vi "View_series_FITS.vi"() -> ()   [LabVIEW 2017] (continued)
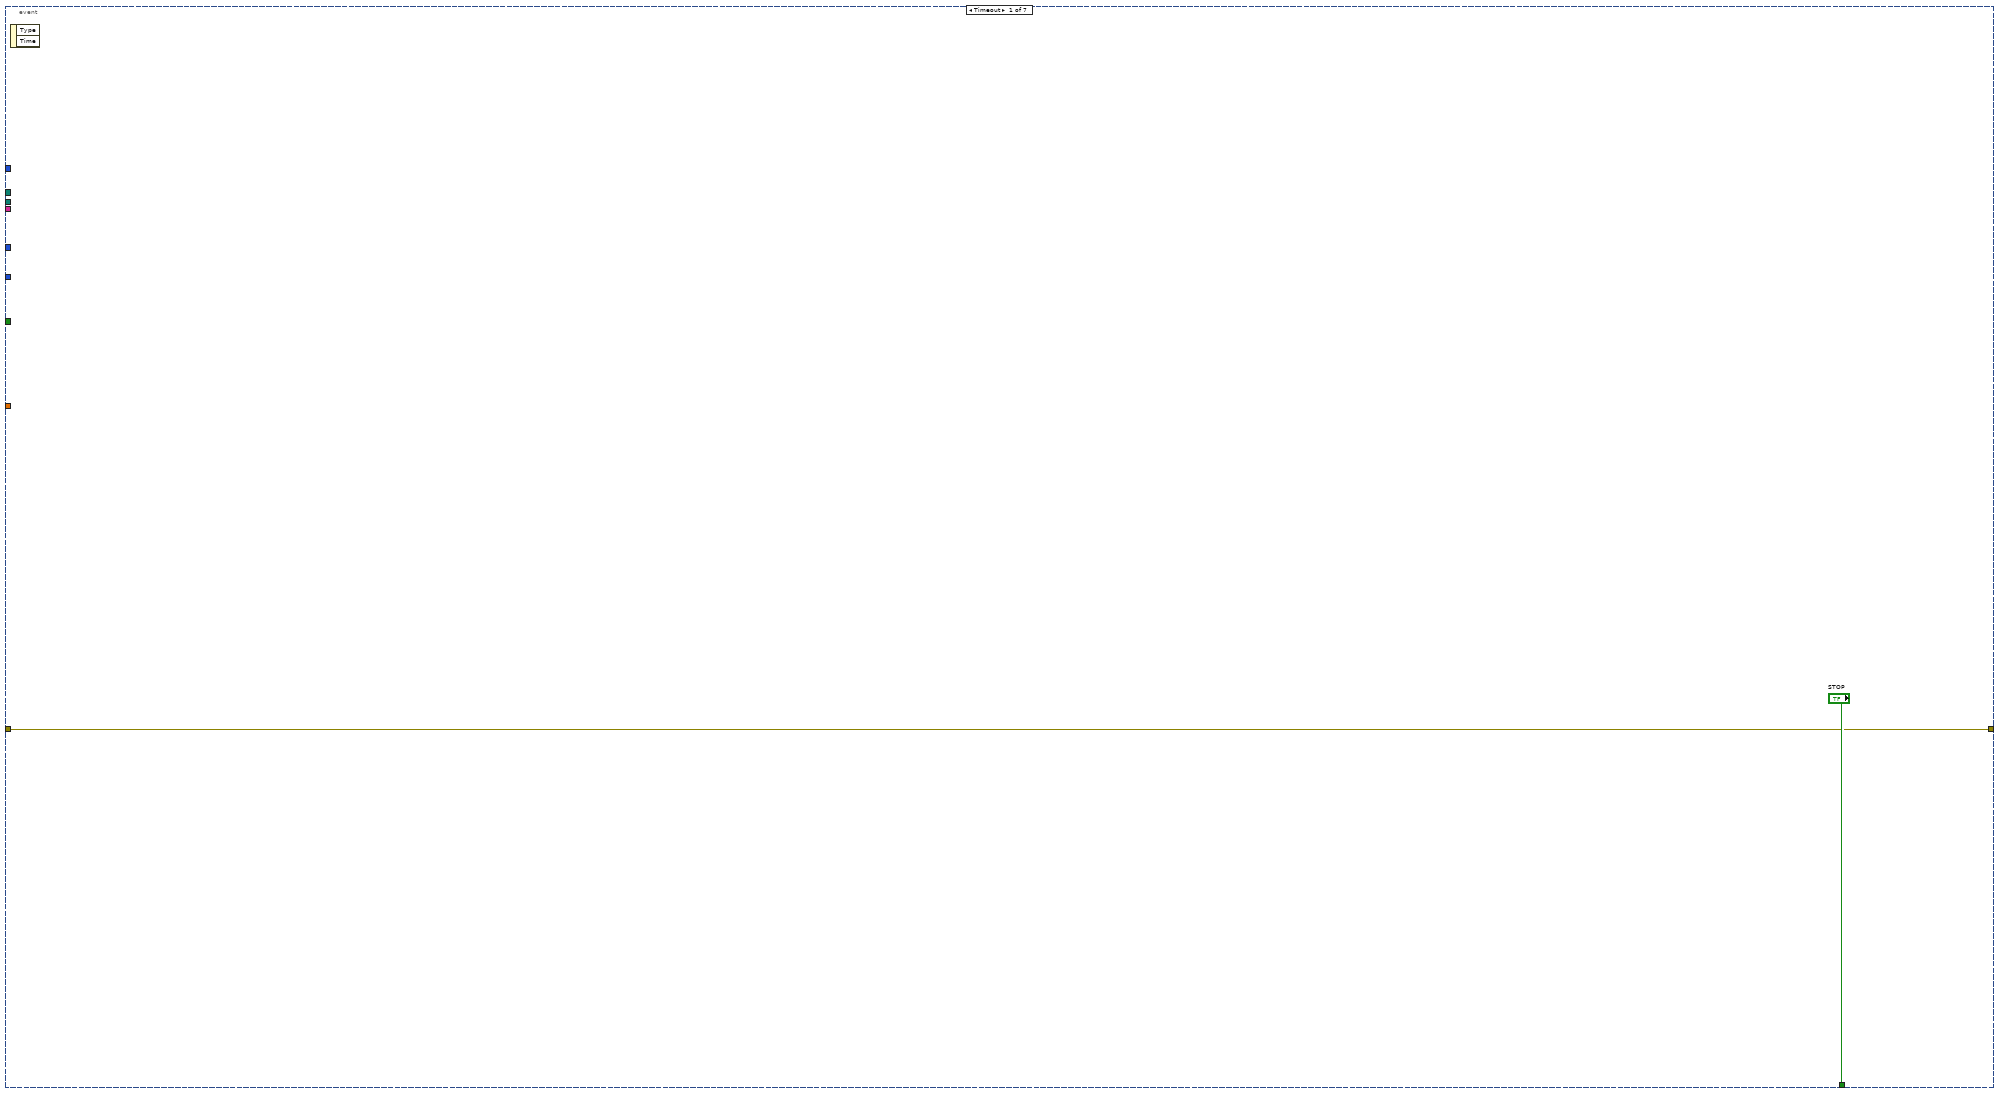
[diagram p3: hidden frame]
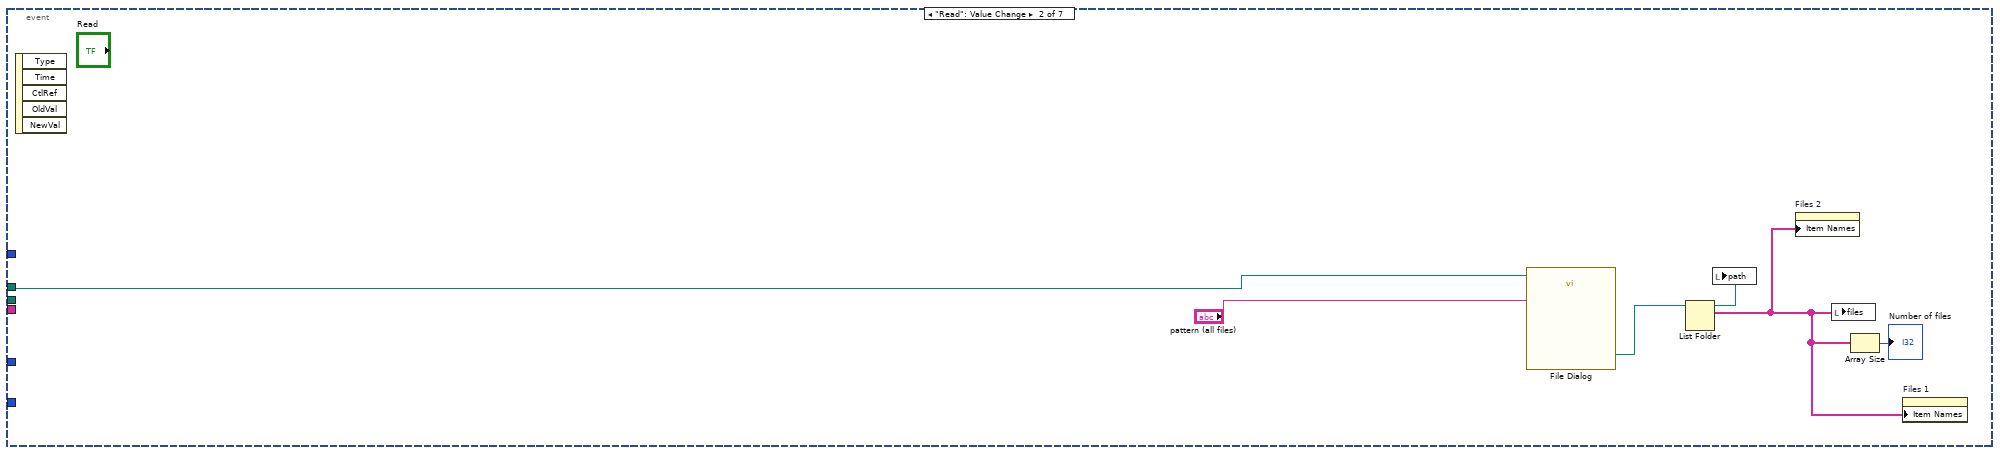
[diagram p4: hidden frame]
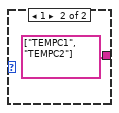
[diagram p5: hidden frame]
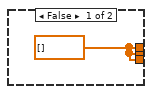
[diagram p11: hidden frame]
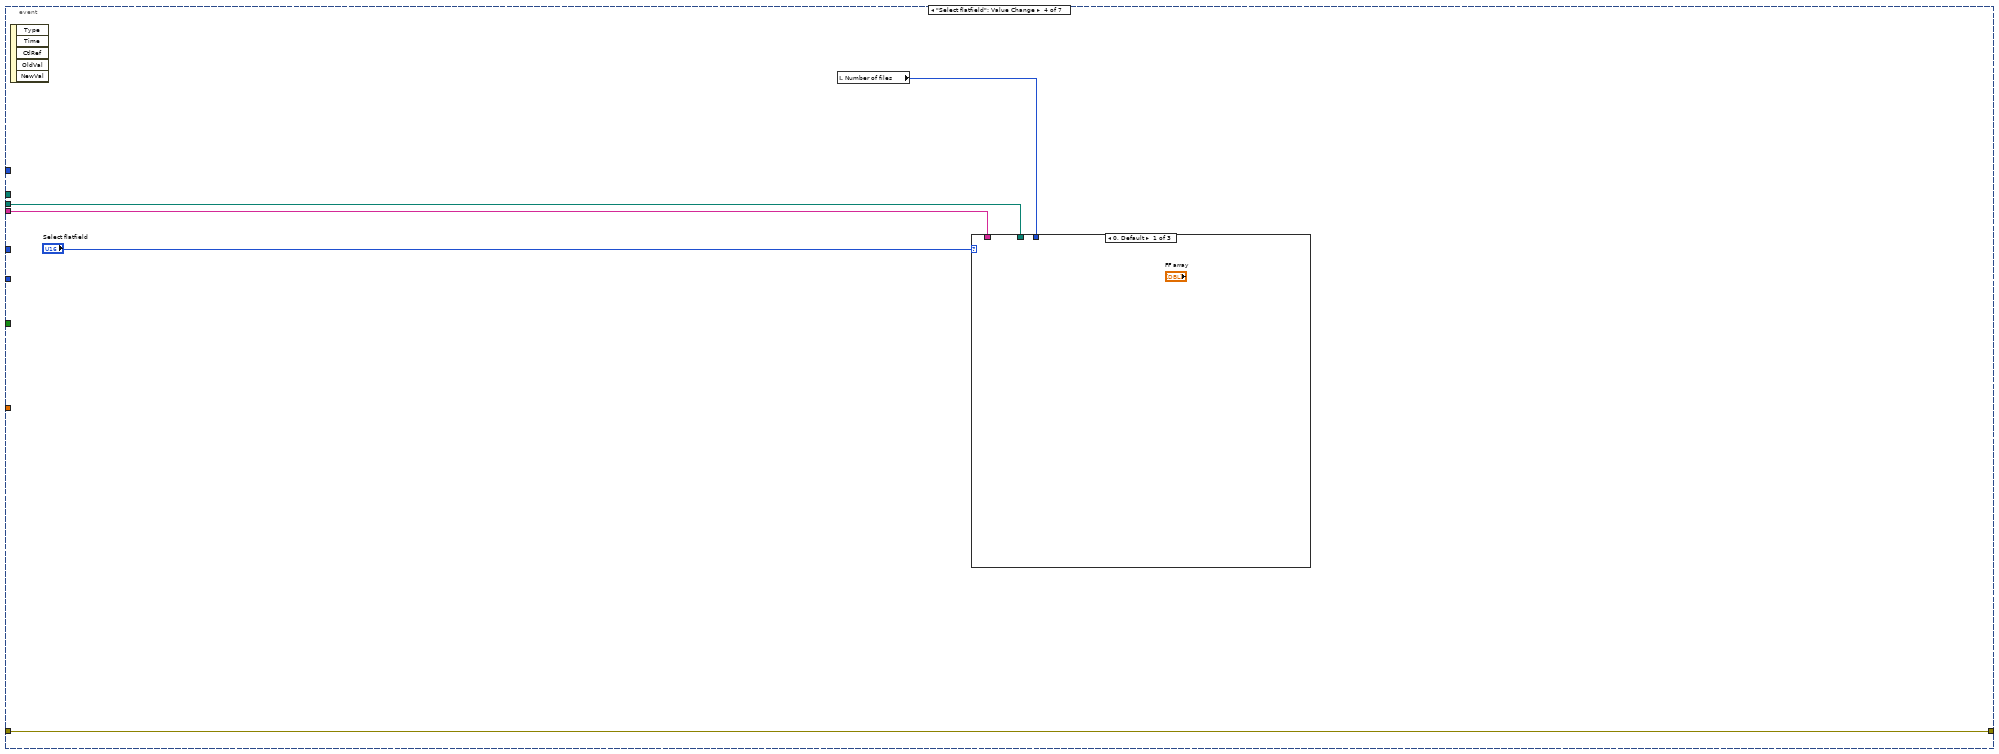
[diagram p14: hidden frame]
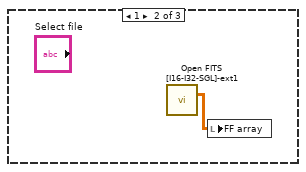
[diagram p15: hidden frame]
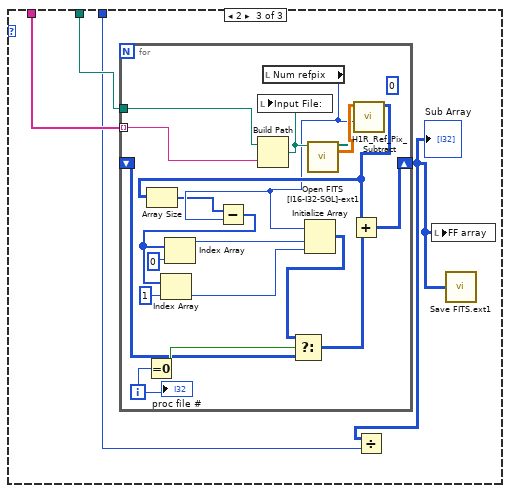
[diagram p16: hidden frame]
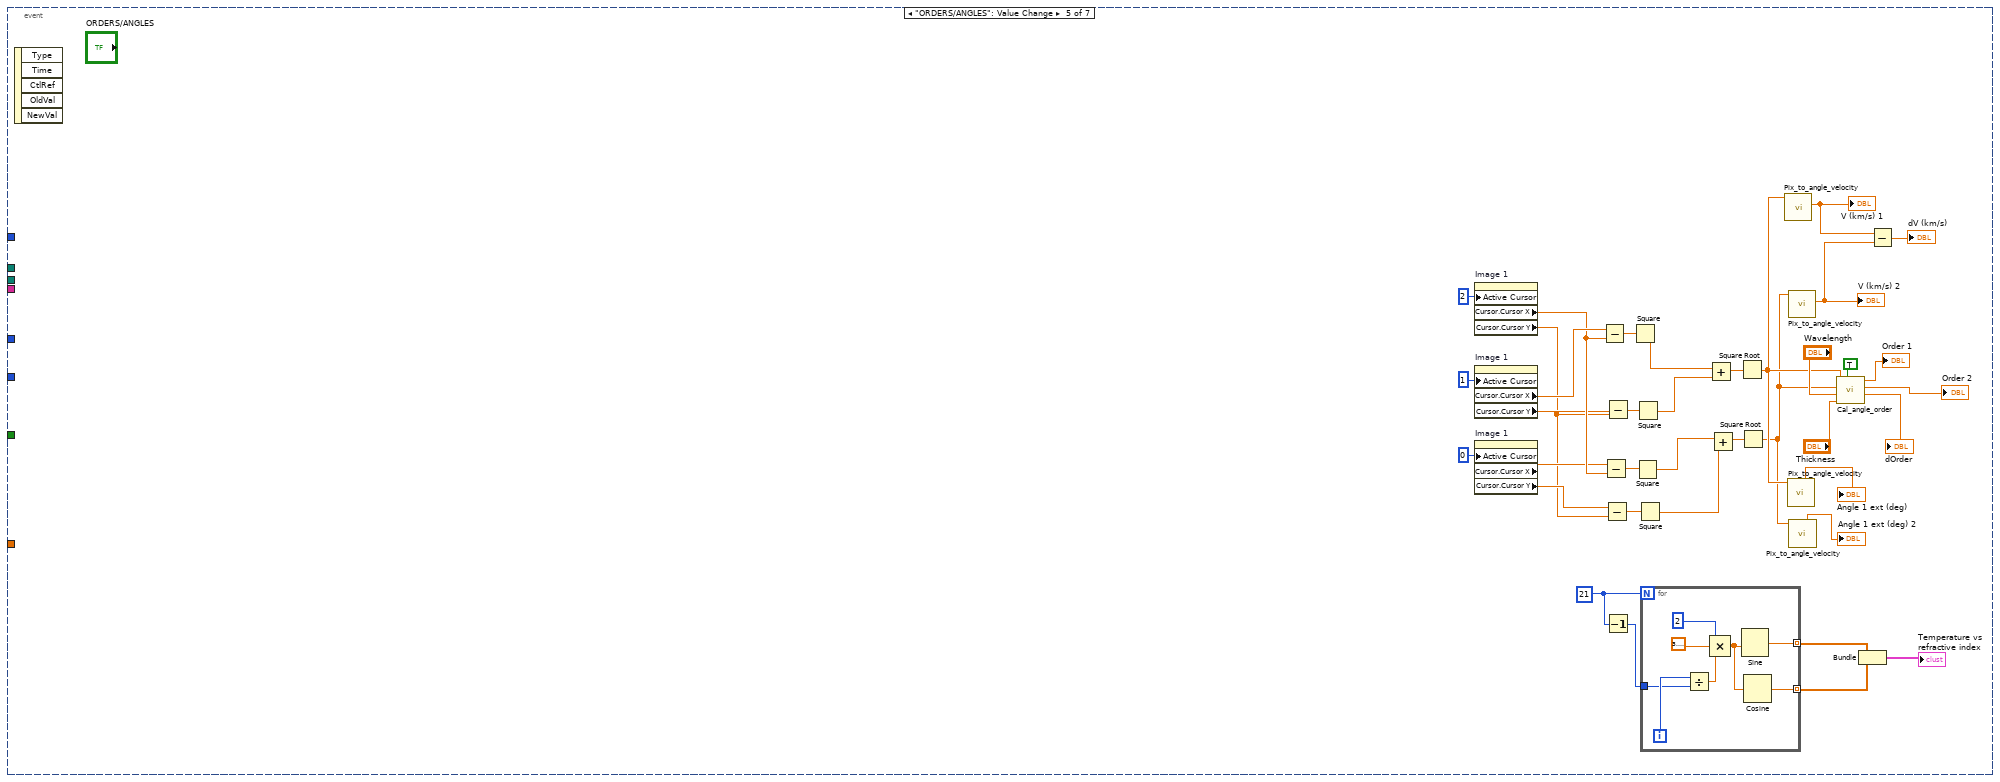
[diagram p17: hidden frame]
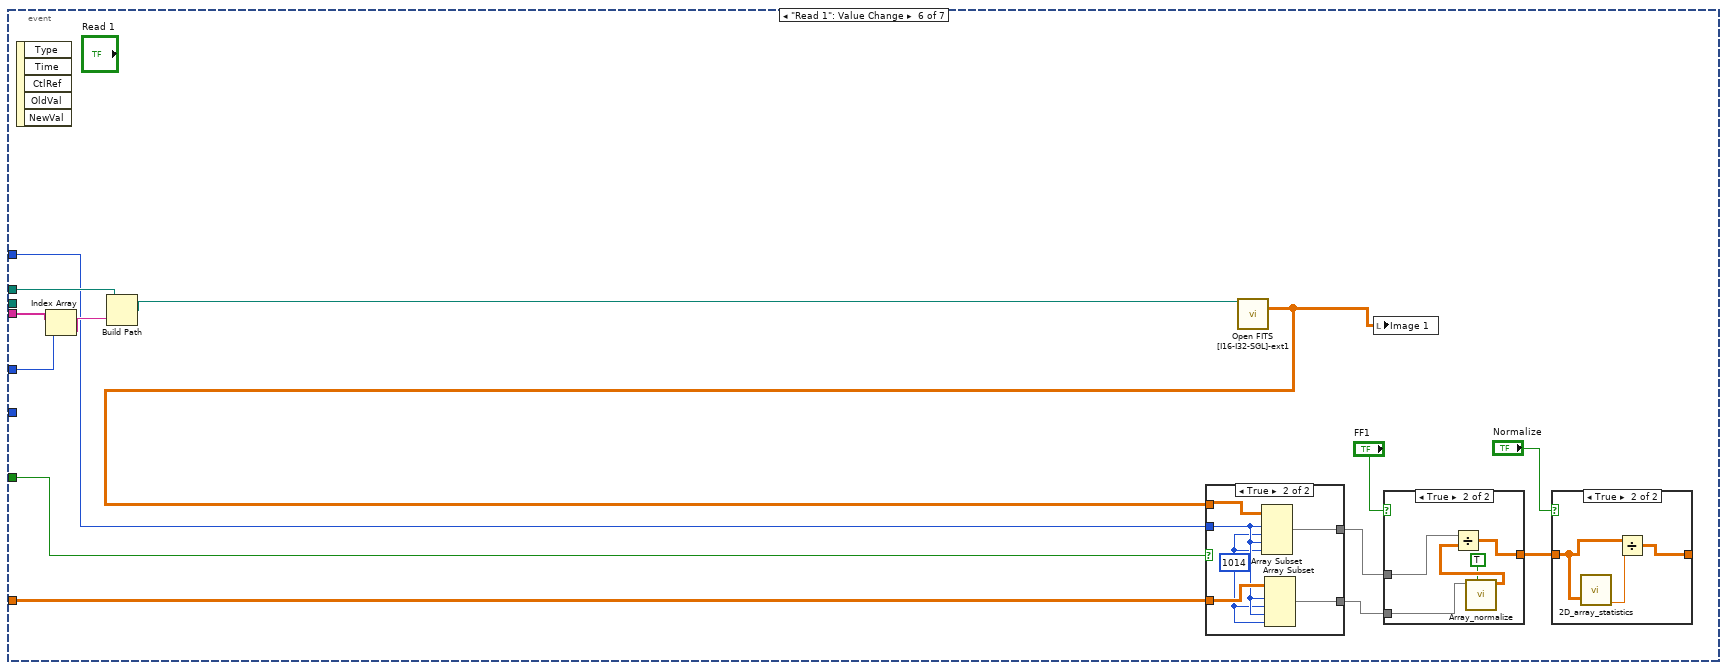
[diagram p18: hidden frame]
              w210 = dbl[] []
            }
            frame True {
              n61 = for {
                N: 4 -> [_]
                tunnel: w216 -> [w227]
                tunnel: [w223] -> w215 mode=indexing
                tunnel: [w222] -> w214 mode=indexing
                tunnel: w211 -> [w220]
                tunnel: [w218] -> w213 mode=indexing
                i -> [w217]
                n62 = property on="Image" class="IntGraph (strict)"("Active Cursor"=w217) -> ("Cursor.Cursor X"=w225:dbl, "Cursor.Cursor Y"=w226:dbl)  [unwired: 2 in, 2 out]
                n63 = call <userlib>:"Sel_arr-Gauss-fit.vi"("parameter bounds"="parameter bounds", "initial guess"=w227, "Cursor.Cursor Y"=w226, "Cursor.Cursor X"=w225, "Selection length"="Selection length", "Sub Array"=w220) -> ("standard deviation"=w222:dbl, "center"=w223:dbl, "amplitude"=w218:dbl, "Slice 2"=→"Slice 2":dbl[])  [unwired: 1 out]
                "STDV" <- w222
                "Amplitude" <- w218
                "Position" <- w223
                "Numeric" <- w217
              }
            }
          }
          n64 = call <userlib>:"FITS_HDR-extr-param.VI"("Header in"=w110, "Param value to write"="INTTIME" ("HDR PARAM name")) -> ("HDR PARAM Value"=w106:dbl)  [unwired: 6 in, 2 out]
          "int tome" <- w106
          n65 = call <userlib>:"DiagnosticsH1R.vi"("Intergation time"=w106, "Array 1"=w89) -> ("Median (ADU/sec)"=w107:dbl)  [unwired: 6 in, 3 out]
          n66 = property on="Image" class="IntGraph (strict)"("Active Cursor"=u32 0) -> ("Cursor.Cursor X"=w155:dbl, "Cursor.Cursor Y"=w152:dbl)  [unwired: 2 in, 2 out]
          n67 = Divide(x=w107, y=w106) -> (x/y=→"Median (ADU/sec)":dbl)
          n68 = Index Array(array=w89, index (col)=w152) -> ()  [unwired: 1 in, 1 out]
          n69 = Index Array(array=w89, index (row)=w155) -> (element=w146:dbl[])  [unwired: 1 in]
          "Slice 4" <- w146
          n70 = local read "file name proc"() -> (w93:string)
          n71 = call <vilib>:"Check if File or Folder Exists.vi"("path"=w94) -> ("file or folder exists?"=w95:bool)  [unwired: 8 in, 2 out]
          n72 = Build Array (concatenate)(w151, w143) -> (w150:dbl[][])
          "Slice 7" <- w150
          n73 = Build Array (concatenate)(w154, w146) -> (w153:dbl[][])
          "Slice 6" <- w153
          n74 = case shown="False" w95 {
            tunnel: w94 -> [w172 w173]
            tunnel: [w171 w173] -> w92
            frame False {
              n75 = Create Folder(path (use dialog)=w172) -> (created path=w171:path, error out=→"error out 2":errorcluster)  [unwired: 2 in, 1 out]
            }
            frame True {
            }
          }
          n76 = Build Path(base path=w92, name or relative path=w93) -> (appended path=w91:path)
          n77 = local write "Init params colS"(w134) -> ()
          n78 = Index Array(array=w124, index (dim 0)=0 ("index")) -> (element=w115:dbl[][])  [unwired: 2 in]
          "Slice 1" <- w115
          n79 = Index Array(array=w124, index (dim 0)=1 ("index")) -> (element=→"Slice 2":dbl[][])  [unwired: 2 in]
          n80 = Index Array(array=w124, index (dim 0)=2 ("index")) -> (element=→"Slice 3":dbl[][])  [unwired: 2 in]
          n81 = local write "Init params ROW"(w135) -> ()
          n82 = case shown="True" "Autosave" {
            selector: "Autosave" -> [_ w167]
            tunnel: w92 -> [_ w169]
            tunnel: w91 -> [_ _]
            tunnel: w89 -> [_ w168]
            frame False {
            }
            frame True {
              n83 = call "Save FITS.ext1.vi"("Default Save Directory"=w169, "Array"=w168, "Append"=w167) -> ()  [unwired: 8 in, 5 out]
            }
          }
          n84 = Index Array(array=w124, index (dim 0)=3 ("index")) -> (element=→"Slice 4":dbl[][])  [unwired: 2 in]
          n85 = Index Array(array=w115, index (row)=0) -> (element=w113:dbl[])  [unwired: 1 in]
        }
        "Amplitude" <- w57
        "Peak position" <- w58
        "STDV" <- w59
        "STDEV" <- w32
        "Amplitude" <- w36
        "STDEV" <- w49
        "center" <- w53
        "Amplitude 2" <- w37
        "STDEV 2" <- w48
        "center 2" <- w52
        "FOCUS" <- w43
        n86 = Build Array("Rows sel", "Cols  sel") -> ()  [unwired: 1 out]
        n87 = Transpose 2D Array(2D array=w43) -> (transposed array=w41:dbl[][])
        n88 = for {
          tunnel: w36 -> [w75]
          tunnel: w37 -> [w70]
          shift-right: [w72] -> w40
          shift-left: dbl[][] [] -> [w74]
          tunnel: "Rows sel" -> [w76] mode=indexing
          tunnel: "Cols  sel" -> [w71] mode=indexing
          i -> [w69]
          n89 = case shown="True" w76 {
            tunnel: w75 -> [_ w86]
            tunnel: [w83 w88] -> w73
            tunnel: w74 -> [w83 w87]
            tunnel: w69 -> [_ w84]
            frame False {
            }
            frame True {
              n90 = Index Array(array=w86, index (col)=w84) -> (element=w85:dbl[])  [unwired: 1 in]
              n91 = Build Array (concatenate)(w87, w85) -> (w88:dbl[][])
            }
          }
          n92 = case shown="True" w71 {
            tunnel: [w77 w82] -> w72
            tunnel: w73 -> [w77 w81]
            tunnel: w70 -> [_ w80]
            tunnel: w69 -> [_ w79]
            frame False {
            }
            frame True {
              n93 = Index Array(array=w80, index (col)=w79) -> (element=w78:dbl[])  [unwired: 1 in]
              n94 = Build Array (concatenate)(w81, w78) -> (w82:dbl[][])
            }
          }
        }
        n95 = for {
          tunnel: w41 -> [w64] mode=indexing
          tunnel: w40 -> [w65]
          tunnel: [w63] -> w42 mode=indexing
          n96 = for {
            tunnel: w65 -> [w66] mode=indexing
            tunnel: w64 -> [w68]
            tunnel: [w67] -> w63 mode=indexing
            n97 = Bundle(w68, w66) -> (w67:cluster{dbl[], dbl[]})  [unwired: 1 in]
            "Array 2" <- w66
          }
          "AXIS 3" <- w63
          "Array" <- w64
        }
        n98 = Index Array(array=w42, index (row)=0) -> (element=→"AXIS 1":cluster{dbl[], dbl[]}[])  [unwired: 1 in]
        n99 = Transpose 2D Array(2D array=w40) -> (transposed array=→"STDEV selected":dbl[][])
      }
      event "Select flatfield": Value Change {
        n100 = event-data() -> ()  [unwired: 1 in, 5 out]
        n101 = local read "Number of files"() -> (w240:i32)
        n102 = case shown="0, Default" "Select flatfield" {
          tunnel: w241 -> [_ _ w247]
          tunnel: w242 -> [_ _ w246]
          tunnel: w240 -> [_ _ w245]
          frame 0, Default {
          }
          frame 1 {
            n103 = call "Open FITS [I16-I32-SGL]-ext1.vi"() -> ("Image"=w243:sgl[][])  [unwired: 11 in, 4 out]
            n104 = local write "FF array"(w243) -> ()
          }
          frame 2 {
            (unwired) 0
            n105 = for {
              tunnel: w247 -> [w264]
              tunnel: w246 -> [w261] mode=indexing
              shift-right: [w263] -> w244
              shift-left: _ -> [w251]
              i -> [w260]
              n106 = Equal To 0?(x=w260) -> (x = 0?=w259:bool)
              n107 = Build Path(base path=w264, name or relative path=w261) -> (appended path=w265:path)
              n108 = local write "Input File:"(w265) -> ()
              n109 = local read "Num refpix"() -> (w250:u16)
              n110 = call "Open FITS [I16-I32-SGL]-ext1.vi"("Input File:"=w265) -> ("Image"=w262:sgl[][])  [unwired: 10 in, 4 out]
              n111 = call <userlib>:"H1R_Ref_Pix_Subtract.vi"("Num Ref Pix"=w250, "Orig Array"=w262) -> ("Sub Array"=w257:i32[][])  [unwired: 9 in]
              n112 = Array Size(array=w257) -> (size(s)=w249:i32[])
              n113 = Subtract(x=w249, y=w250) -> (x-y=w248:i32[])
              n114 = Index Array(array=w248, index=1) -> (element=w253:i32)
              n115 = Index Array(array=w248, index=i16 0 ("element")) -> (element=w254:i32)
              n116 = Initialize Array(w250, w254, w253) -> (w252:u16[][])
              n117 = Select(t=w252, s=w259, f=w251) -> (s? t:f=w258:i32[][])
              n118 = Add(x=w257, y=w258) -> (x+y=w263:i32[][])
              "proc file #" <- w260
            }
            "Sub Array" <- w244
            n119 = Divide(x=w244, y=w245) -> ()  [unwired: 1 out]
            n120 = local write "FF array"(w244) -> ()
            n121 = call "Save FITS.ext1.vi"("Array"=w244) -> ()  [unwired: 10 in, 5 out]
          }
        }
      }
      event "ORDERS/ANGLES": Value Change {
        w277 = 21 ("y")
        n122 = event-data() -> ()  [unwired: 1 in, 5 out]
        n123 = property on="Image 1" class="IntGraph (strict)"("Active Cursor"=u32 2) -> ("Cursor.Cursor X"=w298:dbl, "Cursor.Cursor Y"=w283:dbl)  [unwired: 2 in, 2 out]
        n124 = property on="Image 1" class="IntGraph (strict)"("Active Cursor"=u32 1) -> ("Cursor.Cursor X"=w299:dbl, "Cursor.Cursor Y"=w295:dbl)  [unwired: 2 in, 2 out]
        n125 = property on="Image 1" class="IntGraph (strict)"("Active Cursor"=u32 0) -> ("Cursor.Cursor X"=w297:dbl, "Cursor.Cursor Y"=w296:dbl)  [unwired: 2 in, 2 out]
        n126 = Subtract(x=w299, y=w298) -> (x-y=w294:dbl)
        n127 = Subtract(x=w297, y=w298) -> (x-y=w292:dbl)
        n128 = Subtract(x=w296, y=w283) -> (x-y=w291:dbl)
        n129 = Subtract(x=w295, y=w283) -> (x-y=w293:dbl)
        n130 = Decrement(x=w277) -> (x-1=w276:i32)
        n131 = Square(x=w294) -> (x^2=w290:dbl)
        n132 = Square(x=w292) -> (x^2=w278:dbl)
        n133 = Square(x=w293) -> (x^2=w279:dbl)
        n134 = Square(x=w291) -> (x^2=w289:dbl)
        n135 = for {
          N: w277 -> [_]
          tunnel: w276 -> [w309]
          tunnel: [w306] -> w275 mode=indexing
          tunnel: [w305] -> w274 mode=indexing
          i -> [w310]
          n136 = Divide(x=w310, y=w309) -> (x/y=w308:dbl)
          n137 = Compound Arithmetic op=MULTIPLY(u32 2 ("Active Cursor"), 3.141592653589793, w308) -> (w307:dbl)
          n138 = Sine(x=w307) -> (sin(x)=w306:dbl)
          n139 = Cosine(x=w307) -> (cos(x)=w305:dbl)
        }
        n140 = Add(x=w290, y=w279) -> (x+y=w288:dbl)
        n141 = Add(x=w278, y=w289) -> (x+y=w287:dbl)
        n142 = Square Root(x=w288) -> (sqrt(x)=w269:dbl)
        n143 = Square Root(x=w287) -> (sqrt(x)=w268:dbl)
        n144 = call <userlib>:"Pix_to_angle_velocity.vi"("Pixel distance from cntr"=w269) -> ("V (km/s)"=w272:dbl)  [unwired: 8 in, 2 out]
        "V (km/s) 1" <- w272
        n145 = call <userlib>:"Pix_to_angle_velocity.vi"("Pixel distance from cntr"=w269) -> ("Angle in ext (deg)"=→"Angle 1 ext (deg)":dbl)  [unwired: 8 in, 2 out]
        n146 = call <userlib>:"Pix_to_angle_velocity.vi"("Pixel distance from cntr"=w268) -> ("V (km/s)"=w271:dbl)  [unwired: 8 in, 2 out]
        "V (km/s) 2" <- w271
        n147 = call <userlib>:"Pix_to_angle_velocity.vi"("Pixel distance from cntr"=w268) -> ("Angle in ext (deg)"=→"Angle 1 ext (deg) 2":dbl)  [unwired: 8 in, 2 out]
        n148 = call <userlib>:"Cal_angle_order.vi"("Deg/pixels?"=TRUE, "Thickness"="Thickness", "Wavelength"="Wavelength", "Angle 2 (deg)"=w268, "Angle 1  (deg)"=w269) -> ("dOrder"=→"dOrder":dbl, "Order 2"=→"Order 2":dbl, "Order 1"=→"Order 1":dbl)  [unwired: 4 in]
        n149 = Bundle(w275, w274) -> (→"Temperature vs refractive index":cluster{dbl[], dbl[]})  [unwired: 1 in]
        n150 = Subtract(x=w272, y=w271) -> (x-y=→"dV (km/s)":dbl)
      }
      event "Read 1": Value Change {
        n151 = event-data() -> ()  [unwired: 1 in, 5 out]
        n152 = Index Array(array=w323, index=w322) -> (element=w321:string)
        n153 = Build Path(base path=w324, name or relative path=w321) -> (appended path=w320:path)
        n154 = call "Open FITS [I16-I32-SGL]-ext1.vi"("Input File:"=w320) -> ("Image"=w311:sgl[][])  [unwired: 10 in, 4 out]
        n155 = case shown="True" w315 {
          tunnel: w311 -> [w329 w336]
          tunnel: w317 -> [_ w334]
          tunnel: w318 -> [w330 w335]
          tunnel: [w330 w332] -> w319
          tunnel: [w329 w331] -> w316
          frame False {
          }
          frame True {
            w333 = 1014 ("index")
            n156 = Array Subset(array=w336, index (row)=w334, length (row)=w333, index (col)=w334, length (col)=w333) -> (w331:sgl[][])
            n157 = Array Subset(array=w335, index (row)=w334, length (row)=w333, index (col)=w334, length (col)=w333) -> (w332:dbl[][])
          }
        }
        n158 = local write "Image 1"(w311) -> ()
        n159 = case shown="True" "FF1" {
          tunnel: w316 -> [w337 w342]
          tunnel: [w337 w341] -> w313
          tunnel: w319 -> [_ w338]
          frame False {
          }
          frame True {
            n160 = call <userlib>:"Array_normalize.vi"("Norm?"=TRUE, "Array"=w338) -> ("Array out"=w340:dbl[][])  [unwired: 9 in]
            n161 = Divide(x=w342, y=w340) -> (x/y=w341:dbl[][])
          }
        }
        n162 = case shown="True" "Normalize" {
          tunnel: w313 -> [w325 w328]
          tunnel: [w325 w326] -> _
          frame False {
          }
          frame True {
            n163 = call <userlib>:"2D_array_statistics.vi"("Array"=w328) -> ("median 3"=w327:dbl)  [unwired: 2 in, 3 out]
            n164 = Divide(x=w328, y=w327) -> (x/y=w326:dbl[][])
          }
        }
      }
      event "Read 2": Value Change {
        n165 = event-data() -> ()  [unwired: 1 in, 5 out]
        n166 = Index Array(array=w353, index=w351) -> (element=w355:string)
        n167 = Build Path(base path=w352, name or relative path=w355) -> (appended path=w354:path)
        n168 = call "Open FITS [I16-I32-SGL]-ext1.vi"("Input File:"=w354) -> ("Image"=w348:sgl[][])  [unwired: 10 in, 4 out]
        n169 = case shown="True" w343 {
          tunnel: w348 -> [w356 w363]
          tunnel: w346 -> [_ w361]
          tunnel: w347 -> [w357 w362]
          tunnel: [w357 w359] -> w350
          tunnel: [w356 w358] -> w349
          frame False {
          }
          frame True {
            w360 = 1014 ("index")
            n170 = Array Subset(array=w363, index (row)=w361, length (row)=w360, index (col)=w361, length (col)=w360) -> (w358:sgl[][])
            n171 = Array Subset(array=w362, index (row)=w361, length (row)=w360, index (col)=w361, length (col)=w360) -> (w359:dbl[][])
          }
        }
        n172 = case shown="True" "FF2" {
          tunnel: w349 -> [w364 w369]
          tunnel: [w364 w368] -> w345
          tunnel: w350 -> [_ w365]
          frame False {
          }
          frame True {
            n173 = call <userlib>:"Array_normalize.vi"("Norm?"=TRUE, "Array"=w365) -> ("Array out"=w367:dbl[][])  [unwired: 9 in]
            n174 = Divide(x=w369, y=w367) -> (x/y=w368:dbl[][])
          }
        }
        "Image 2" <- w345
      }
    }
  }
